vi "Python.vi"(8 "error in (no error)":errorcluster) -> (0 "error out":errorcluster, 3 "BinCache":path)   [LabVIEW 2013, in "Advanced Plotting Toolkit.lvlib"]
uses:
  Advanced Plotting Toolkit.lvlib
  <vilib>/Utility/sysdir.llb/System Directory Type.ctl
  <vilib>/zip/NI_Unzip.lvlib
panel:
  in  "FolderKey":string="debug"
  in  "Data":u8[](array[numeric])=array[4936996 elements]
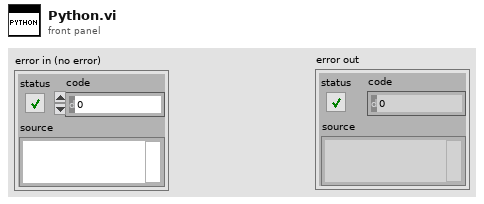
[diagram p1: front panel]
types:
  T1 = typedef "System Directory Type.ctl" = i32
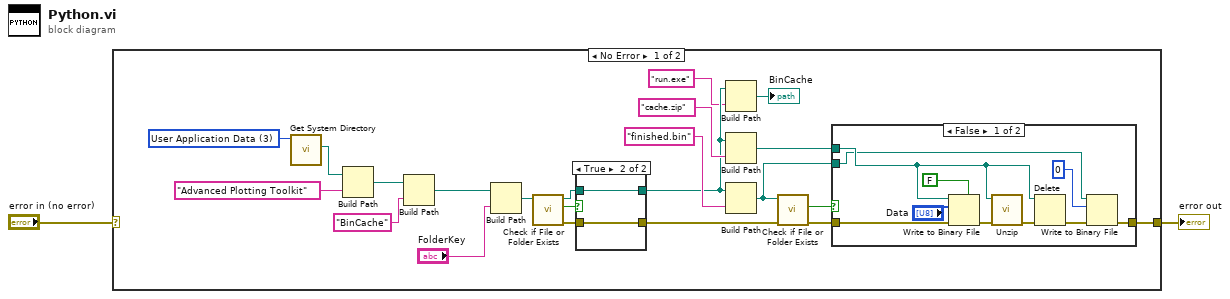
[diagram p0: block diagram]
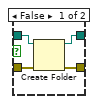
[diagram p3: hidden frame]
diagram:
  n1 = case shown="No Error" "error in (no error)" {
    selector: "error in (no error)" -> [_ w42]
    tunnel: [w3 w42] -> w1
    frame No Error {
      w24 = T1 3 items=["User Home"=0, "User Desktop"=1, "User Documents"=2, "User Application Data"=3, "User Preferences"=4, "User Temporary"=5, "Public Documents"=6, "Public Application Data"=7, "Public Preferences"=8, "Public Cache"=13, "System Core Libraries"=9, "System Installed Libraries"=10, "Application Files"=11, "Boot Volume Root"=12] ("system directory type")
      n2 = call <vilib>:"Get System Directory.vi"("system directory type"=w24) -> ("system directory"=w23:path)  [unwired: 10 in]
      n3 = Build Path(base path=w23, name or relative path="Advanced Plotting Toolkit") -> (appended path=w21:path)
      n4 = Build Path(base path=w21, name or relative path="BinCache") -> (appended path=w18:path)
      n5 = Build Path(base path=w18, name or relative path="FolderKey") -> (appended path=w17:path)
      n6 = call <vilib>:"Check if File or Folder Exists.vi"("path"=w17) -> ("error out"=w6:errorcluster, "file or folder exists?"=w16:bool, "dup path"=w15:path)  [unwired: 8 in]
      n7 = case shown="True" w16 {
        tunnel: w15 -> [w39 w41]
        tunnel: [w38 w41] -> w9
        tunnel: w6 -> [w37 w40]
        tunnel: [w36 w40] -> w5
        frame False {
          n8 = Create Folder(path (use dialog)=w39, error in=w37) -> (created path=w38:path, error out=w36:errorcluster)  [unwired: 1 in, 1 out]
        }
        frame True {
        }
      }
      n9 = Build Path(base path=w9, name or relative path="run.exe") -> (appended path=→"BinCache":path)
      n10 = Build Path(base path=w9, name or relative path="cache.zip") -> (appended path=w11:path)
      n11 = Build Path(base path=w9, name or relative path="finished.bin") -> (appended path=w10:path)
      n12 = call <vilib>:"Check if File or Folder Exists.vi"("error in (no error)"=w5, "path"=w10) -> ("error out"=w4:errorcluster, "file or folder exists?"=w13:bool)  [unwired: 7 in, 1 out]
      n13 = case shown="False" w13 {
        tunnel: w11 -> [w31 _]
        tunnel: w10 -> [w30 _]
        tunnel: w4 -> [w27 w35]
        tunnel: [w26 w35] -> w3
        frame False {
          n14 = Write to Binary File(file (use dialog)=w31, data="Data", error in=w27, 5:FALSE ("prepend array or string size? (T)")) -> (error out=w33:errorcluster)  [unwired: 2 in, 2 out]
          n15 = call <vilib>:"Unzip.vi"("error in (no error)"=w33, "Zip file"=w31) -> ("error out"=w32:errorcluster)  [unwired: 7 in, 2 out]
          n16 = Delete(path (use dialog)=w31, error in=w32) -> (error out=w28:errorcluster)  [unwired: 3 in, 2 out]
          n17 = Write to Binary File(file (use dialog)=w30, data=u8 0, error in=w28) -> (error out=w26:errorcluster)  [unwired: 3 in, 2 out]
        }
        frame True {
        }
      }
    }
    frame Error {
    }
  }
  "error out" <- w1
